vi "Trajectory Builder.vi"() -> ()   [LabVIEW 2023]
uses:
  Types/Limits.ctl
  Types/Overrides.ctl
  Types/Trajectory Data.ctl
  Types/Segment Type.ctl
  Types/Path Type.ctl
  Types/Drive Type.ctl
  Types/Angluar Limits.ctl
  Types/Command Editor Info.ctl
  Types/Single Cmd Info.ctl
  <vilib>/picture/picture.llb/imagedata.ctl
  <vilib>/Utility/miscctls.llb/LVPositionTypeDef.ctl
  <vilib>/Utility/miscctls.llb/LVRowAndColumnTypeDef.ctl
  Types/Internal Path Stuff.ctl
  <vilib>/Utility/miscctls.llb/LVBoundsTypeDef.ctl
  <vilib>/event_ctls.llb/lveventtype.ctl
  Global Settings.vi
panel:
  in  "Push":bool
  out "Picture":picture
  out "C":bool
  in  "Cache":T4
  out "Trajectory Data":T5
  out "CU":bool
  in  "Zero Velocity":bool
  in  "Reverse Path":bool
  in  "Robot Backwards":bool
  out "Duration (s)":dbl format="%#.4g"
  out "Distance (ft)":dbl format="%#.1g"
  in  "Instructions":string="Directions:\nUse mouse to ...\n    move robot position (rectangle with arrow)\n    rotate robot (red arrow)\n    move waypoints (numbered circles)\nClick in open space to add a waypoint\nShift click to delete a waypoint\nHover over a waypoint and use arrow keys to nudge\n\nTime slider and Play button will run robot along path to test for collisions.\n\nNew creates a new path at default location\n\nAppend creates a path using current path's position and heading.\n\nTo add a command, move robot using Time slider and double click the Command in Palette.\n\nYou can modify command timing in the graph or Command Sequencer tree.\n\nEnable/disable a command by clicking on the enable column item.\n\nDelete a command by shift-clicking in the enable column.\n\nTo configure command parameters, Select the command name in the tree, Open Panel, enter parameters, and Inhale the parameters.\n\nYou may sometimes want to type values into WayPoints directly.\n\nOverrides allow you to set accel and V limits for any turn."
  out "Command Palette":picture
  in  "Directory":bool
  in  "Tab Control":T7(tab)
  in  "Angular Limits":T8={"Velocity (deg/s)"=6.0, "Accel (deg/s^2)"=360.0, "Jerk (deg/s^3)"=1000.0} {"Jerk (deg/s^3)" min=0.01 step=1.0; "Accel (deg/s^2)" min=0.01; "Velocity (deg/s)" min=0.01}
  in  "Path Type":T9=enum."Bezier"
  in  "Overrides":T10=[{"Count"="1", "Angular Override"=0.0, "Enabled?"=FALSE, "Velocity Override"=6.0, "Angle Override"=nan}] {"Angle Override" step=5.0; "Velocity Override" step=5.0; "Angular Override" step=5.0}
  in  "Center Flip":bool
  in  "Sample Period (s)":dbl=0.02 min=0.001 max=1.0 format="%#_6p"
  in  "Limits":T11={"Velocity (fps)"=6.0, "Accel (fps^2)"=15.0, "Jerk (fps^3)"=150.0, "StoopidFast (fps)"=6.0} {"StoopidFast (fps)" min=0.01; "Jerk (fps^3)" min=0.01 step=1.0; "Accel (fps^2)" min=0.01; "Velocity (fps)" min=0.01}
  in  "Conditions":T12 {"vFinal (fps)" min=0.0; "vInitial (fps)" min=0.0}
  in  "Drive Type":T13=enum."Holonomic"
  in  "WayPoints":cluster{"x":dbl, "y":dbl, "th":dbl}[](array[cluster])
  in  "Turn Angle Limit (deg)":dbl=90.0
  in  "Allow Angles > 90":bool=TRUE
  in  "Stoopid Overlap %":dbl min=0.0
  in  "Unjank":bool
  in  "Turn Deceleration":bool=TRUE
  in  "Turn Acceleration":bool=TRUE
  in  "Open Command":bool
  in  "Inhale":bool
  in  "Command Sequence":string(tree)
  in  "Projects":u16(ring) items=["2024 Crescendo Robot Project.lvproj"]
  in  "Refresh":bool
  in  "Snap to foot":bool
  in  "Angle Limiter":enum16{"90", "45", "15", "1"}(ring)=enum."15"
  in  "Snap robot to baseline":bool
  in  "Background":u16(ring) items=["C Field", "CU Field", "RR Field", "IR Field", "Barrels", "Bounce", "Slalom", "Galactic Search A", "Galactic Search B"]
  in  "Robot Color":u32(colorbox)=14421504
  out "Field Size (ft)":cluster{"width":dbl, "height":dbl}={"width"=26.9167, "height"=35.2142} {"width" format="%#.1g"; "height" format="%#.1g"}
  in  "Robot Size (in)":cluster{"width":dbl, "height":dbl}={"width"=28.0, "height"=28.0}
  in  "Hide Path":bool
  in  "Time (s)":dbl(slide) scale=0.0..3.1199999999999997 scale format="%#.1g"
  in  "Play":bool
  out "fps":dbl[](graph)
  in  "Append":bool
  in  "Open":i32(listbox)
  in  "Filename":string
  in  "Save":bool
  in  "New":bool
  out "slalom":bool
  out "barrels":bool
  out "bounce":bool
  out "G-S B":bool
  out "G-S A":bool
  out "RR":bool
  out "IRR":bool
  # "Command Palette"
  # "StupidFast makes each linear segment into a\nvelocity ramp to max speed (for clothoid paths only)"
  # "Nicotine"
  # "A"
  # "V"
  # "O"
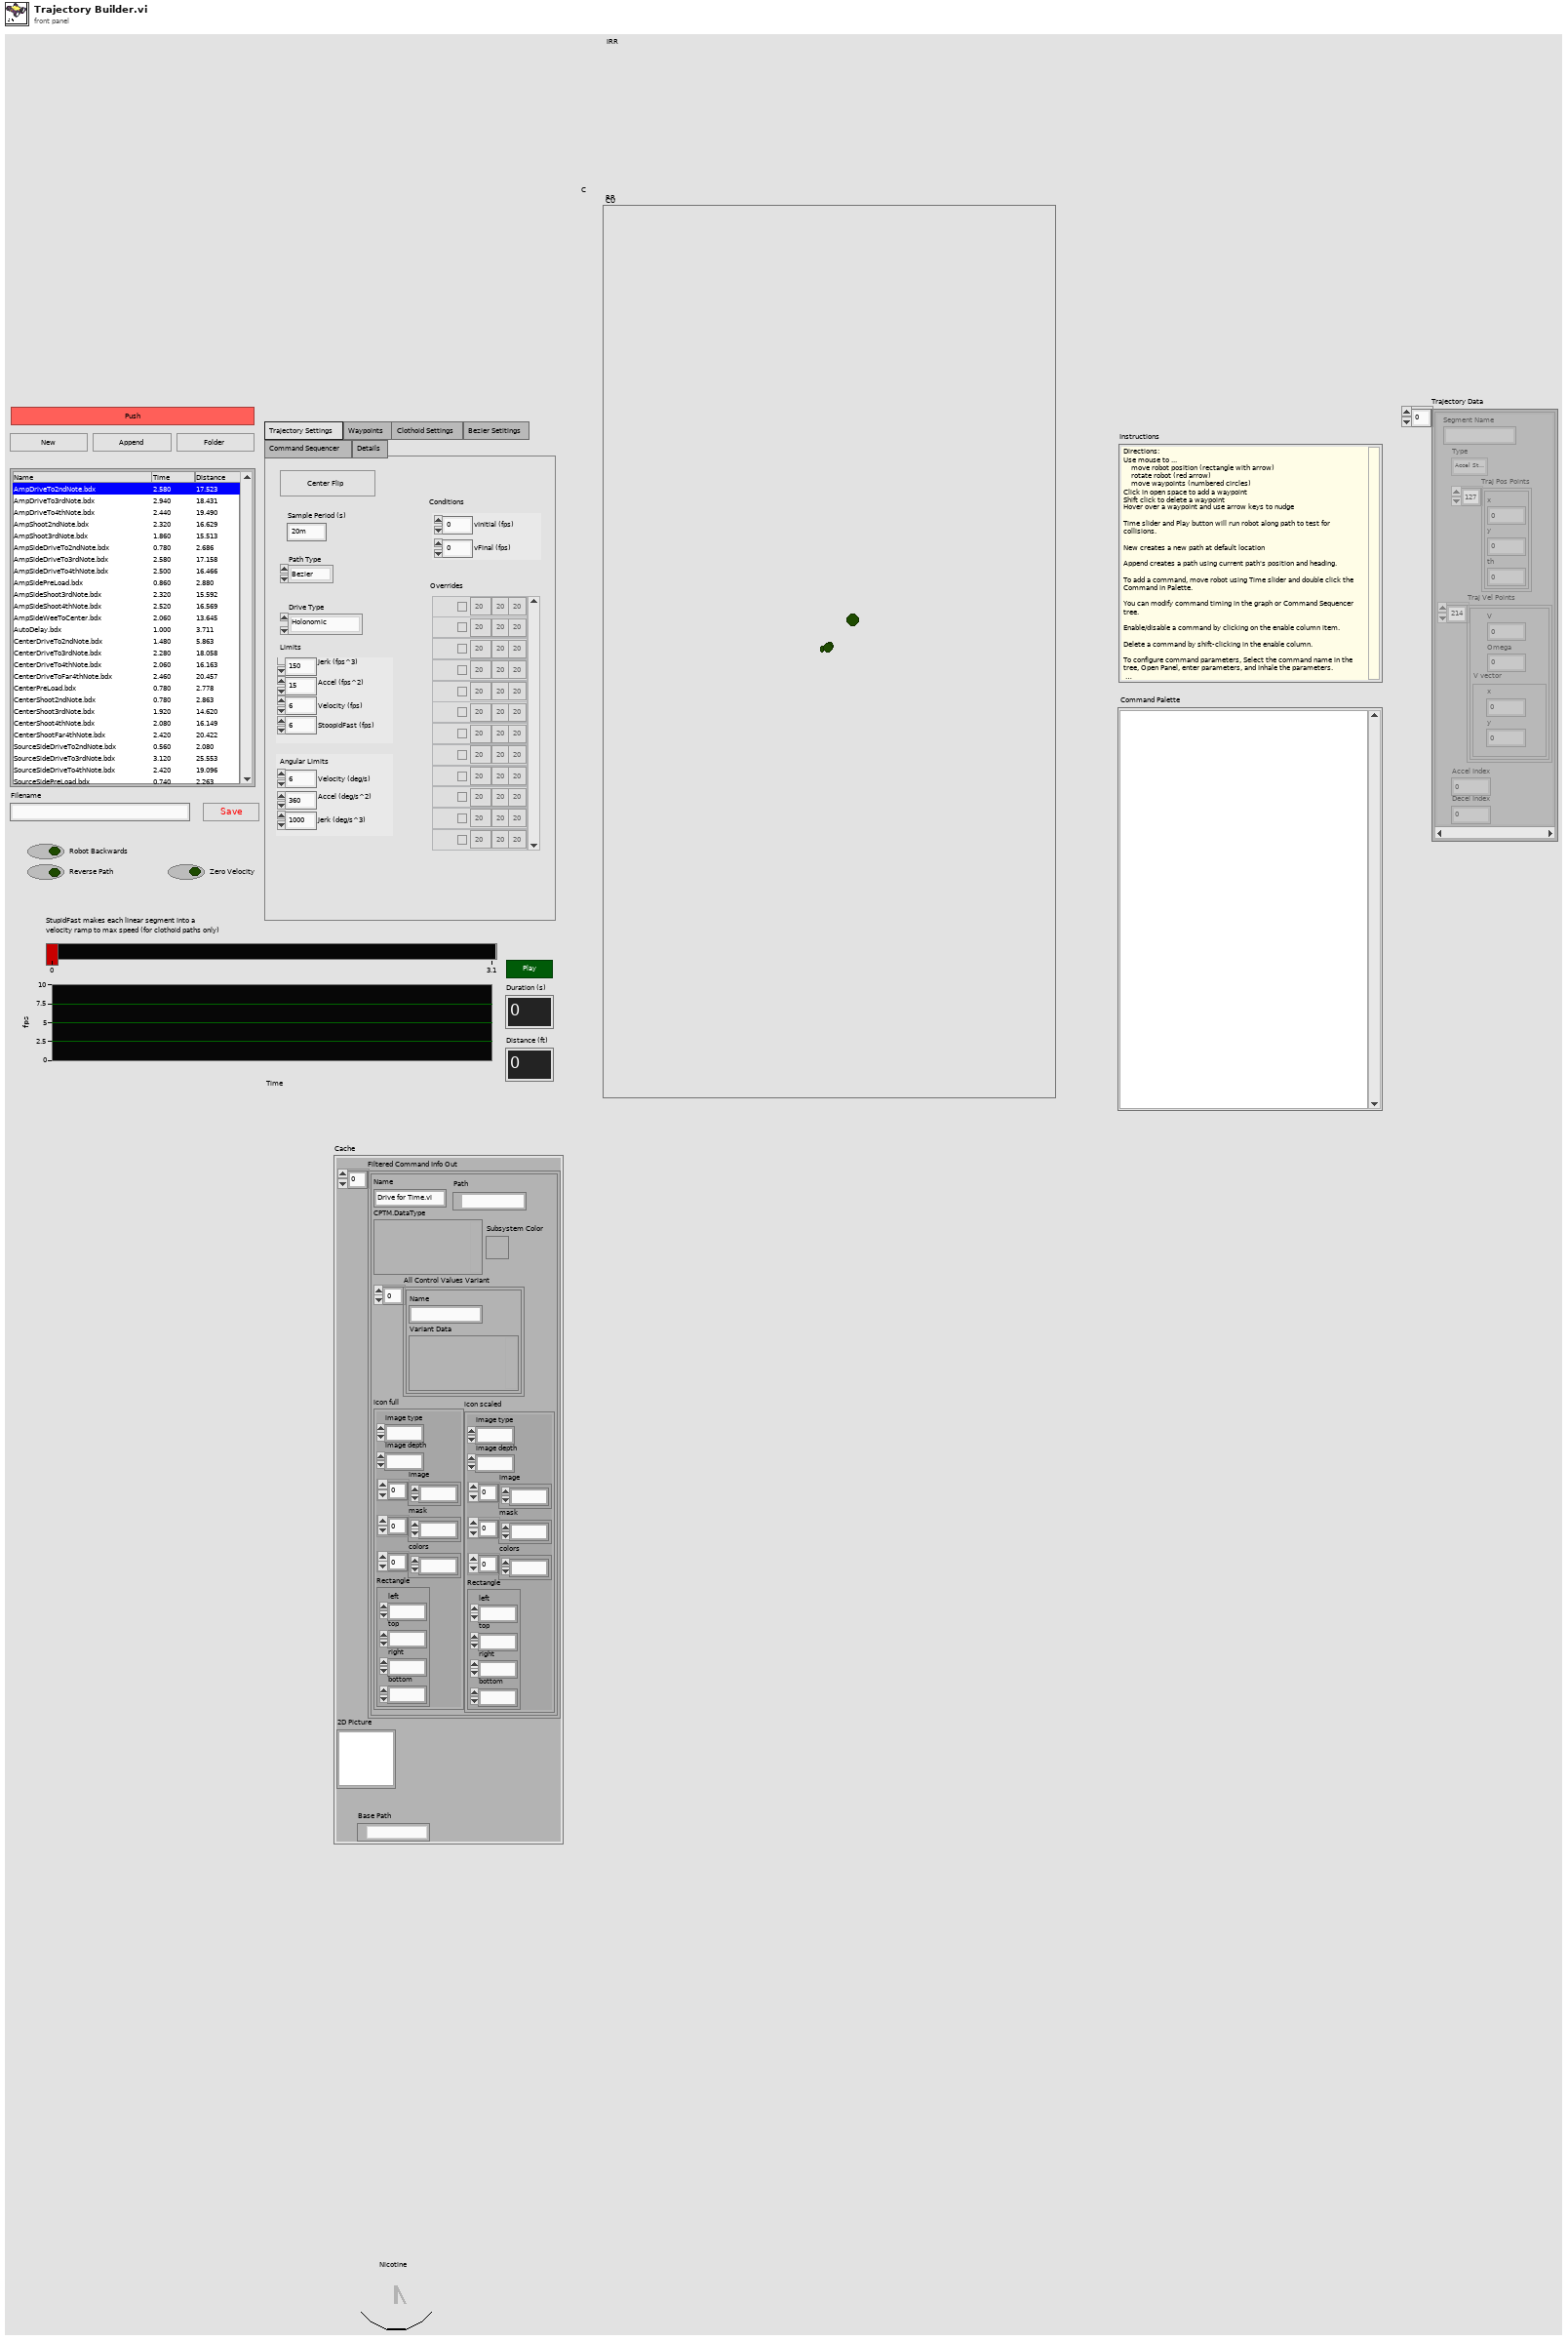
[diagram p1: front panel]
types:
  T1 = typedef "Command Editor Info.ctl" = T2[]
  T2 = typedef "Single Cmd Info.ctl" = cluster{"Name":string, "CPTM.DataType":variant, "All Control Values Variant":cluster{"Name":string, "Variant Data":variant}[], "icon full":T3, "icon scaled":T3, "Path":path, "Subsystem Color":u32}
  T3 = typedef "imagedata.ctl" = cluster{"image type":i32, "image depth":i32, "image":u8[], "mask":u8[], "colors":u32[], "Rectangle":cluster{"left":i16, "top":i16, "right":i16, "bottom":i16}}
  T4 = cluster{"Filtered Command Info Out":T1, "2D Picture":picture, "Base Path":path}
  T5 = typedef "Trajectory Data.ctl" = cluster{"Segment Name":string, "Type":T6, "Traj Pos Points":cluster{"x":dbl, "y":dbl, "th":dbl}[], "Traj Vel Points":cluster{"V":dbl, "Omega":dbl, "V vector":cluster{"y":dbl, "x":dbl}}[], "Accel Index":i32, "Decel Index":i32}[]
  T6 = typedef "Segment Type.ctl" = enum16{"Accel Straight", "Const Straight", "Blend", "Circle", "Bezier"}
  T7 = enum32{"Trajectory Settings", "Waypoints", "Clothoid Settings", "Bezier Setitings", "Command Sequencer", "Details"}
  T8 = typedef "Angluar Limits.ctl" = cluster{"Velocity (deg/s)":dbl, "Accel (deg/s^2)":dbl, "Jerk (deg/s^3)":dbl}
  T9 = typedef "Path Type.ctl" = enum16{"Clothoid", "Bezier"}
  T10 = typedef "Overrides.ctl" = cluster{"Count":string, "Angular Override":dbl, "Enabled?":bool, "Velocity Override":dbl, "Angle Override":dbl}[]
  T11 = typedef "Limits.ctl" = cluster{"Velocity (fps)":dbl, "Accel (fps^2)":dbl, "Jerk (fps^3)":dbl, "StoopidFast (fps)":dbl}
  T12 = cluster{"vInitial (fps)":dbl, "vFinal (fps)":dbl}
  T13 = typedef "Drive Type.ctl" = enum16{"Nonholonomic", "Holonomic"}
  T14 = cluster{"Sample Period (s)":dbl, "Limits":T11, "Conditions":cluster{"vInitial (fps)":dbl, "vFinal (fps)":dbl}, "Overrides":T10, "Angular Limits":T8}
  T15 = typedef "LVRowAndColumnTypeDef.ctl" = cluster{"Row":i32, "Column":i32}
  T16 = typedef "LVPositionTypeDef.ctl" = cluster{"Left":i32, "Top":i32}
  T17 = cluster{"Index":i32, "Pt Test Results":enum16{"Miss", "Rect Hit", "Arrow Hit"}}
  T18 = cluster{"Drag Object":cluster{"Index":i32, "x":dbl, "y":dbl}, "Hover Object":cluster{"Index":i32, "Pt Test Results":enum16{"Miss", "Rect Hit", "Arrow Hit"}}, "Filename":string}
  T19 = cluster{"Trajectory Data":T5, "Points":cluster{"x":dbl, "y":dbl, "th":dbl}[], "output cluster":cluster{"Sample Period (s)":dbl, "Limits":T11, "Conditions":cluster{"vInitial (fps)":dbl, "vFinal (fps)":dbl}, "Overrides":T10, "Angular Limits":T8}, cluster{"Time (s)":dbl, T2, bool}[]}
  T20 = typedef "Internal Path Stuff.ctl" = cluster{"Trajectory Data":T5, "Updated Waypoints":cluster{"x":dbl, "y":dbl, "th":dbl}[], cluster{"Sample Period (s)":dbl, "Limits":T11, "Conditions":cluster{"vInitial (fps)":dbl, "vFinal (fps)":dbl}, "Overrides":T10, "Angular Limits":T8}, "Commands out":cluster{"Time (s)":dbl, T2, bool}[]}
  T21 = typedef "LVBoundsTypeDef.ctl" = cluster{"Width":u32, "Height":u32}
  T22 = typedef "lveventtype.ctl" = enum32{"Null", "Timeout", "Annotation Menu Selection", "Annotation Menu Selection?", "App Instance Close", "App Instance Close?", "Autoscale Range Change", "Bookmark Info Change", "Cell Edit", "Cell Edit?", "Cursor Grab", "Cursor Grab?", "Cursor Menu Selection", "Cursor Menu Selection?", "Cursor Move", "Cursor Release", "Data Change", "Direction Change", "Display State Change", "Drag Ended", "Drag Enter", "Drag Leave", "Drag Over", "Drag Source Update", "Drag Starting", "Drag Starting?", "Drop", "Exec State Change", "Key Down", "Key Down?", "Key Repeat", "Key Repeat?", "Key Up", "Listbox Double Click", "Menu Activation?", "Menu Selection (App)", "Menu Selection? (App)", "Menu Selection (User)", "Mouse Down", "Mouse Down?", "Mouse Enter", "Mouse Leave", "Mouse Move", "Mouse Up", "Mouse Wheel", "NI Security User Change (App)", "Pane Size", "Panel Close", "Panel Close?", "Panel Resize", "Plot Attribute Change", "Scale Range Change", "Shortcut Menu Activation?", "Shortcut Menu Selection (App)", "Shortcut Menu Selection? (App)", "Shortcut Menu Selection (User)", "Tree Double Click", "Tree Drag", "Tree Drag?", "Tree Drop", "Tree Drop?", "Tree Item Close", "Tree Item Close?", "Tree Item Open", "Tree Item Open?", "User Event", "Value Change"}
  T23 = enum32{"Invalid", "Standard", "Closed", "Hidden", "Minimized", "Maximized"}
  T24 = cluster{"width":dbl, "height":dbl, "width":dbl, "height":dbl}
  T25 = cluster{"Robot Backwards":bool, "Reverse Path":bool}
  T26 = cluster{cluster{"Robot Backwards":bool, "Reverse Path":bool}, "Trajectory Data":T5, "Commands out":cluster{"Time (s)":dbl, T2, bool}[], cluster{"Sample Period (s)":dbl, "Limits":T11, "Conditions":cluster{"vInitial (fps)":dbl, "vFinal (fps)":dbl}, "Overrides":T10, "Angular Limits":T8}, "Updated Waypoints":cluster{"x":dbl, "y":dbl, "th":dbl}[], "Time & Dist":cluster{"Time (s)":dbl, "Distance (ft)":dbl}, "Zero Velocity":bool, cluster{"Drive Type":T13, "Path Type":T9}}
  T27 = cluster{"Trajectory Data":T5, "Updated Waypoints":cluster{"x":dbl, "y":dbl, "th":dbl}[], cluster{"Sample Period (s)":dbl, "Limits":T11, "Conditions":cluster{"vInitial (fps)":dbl, "vFinal (fps)":dbl}, "Overrides":T10, "Angular Limits":T8}, "Commands out":cluster{"Time (s)":dbl, T2, bool}[]}
  T28 = cluster{"Sample Period (s)":dbl, cluster{"Velocity (fps)":dbl, "Accel (fps^2)":dbl, "Jerk (fps^3)":dbl, "StoopidFast (fps)":dbl}, "Conditions":cluster{"vInitial (fps)":dbl, "vFinal (fps)":dbl}, "Overrides":T10, "Angular Limits":T8}
  T29 = cluster{"Velocity (fps)":dbl, "Accel (fps^2)":dbl, "Jerk (fps^3)":dbl, "StoopidFast (fps)":dbl}
  T30 = cluster{"Trajectory Data":T5, "Points out":cluster{"x":dbl, "y":dbl, "th":dbl}[], "Fields":cluster{"Sample Period (s)":dbl, cluster{"Velocity (fps)":dbl, "Accel (fps^2)":dbl, "Jerk (fps^3)":dbl, "StoopidFast (fps)":dbl}, "Conditions":cluster{"vInitial (fps)":dbl, "vFinal (fps)":dbl}, "Overrides":T10, "Angular Limits":T8}, "Commands out":cluster{"Time (s)":dbl, T2, bool}[]}
  T31 = typedef "LVPoint32TypeDef.ctl" = cluster{"Horizontal":i32, "Vertical":i32}
  T32 = cluster{"Shift":bool, "Ctrl":bool, "Alt":bool, "Cmd":bool, "Opt":bool}
  T33 = cluster{"Snap robot to baseline":bool, "Snap to foot":bool, "Angle Limiter":enum16{"90", "45", "15", "1"}}
  T34 = cluster{i32, "Pt Test Results":enum16{"Miss", "Rect Hit", "Arrow Hit"}}
  T35 = typedef "eventvkey.ctl" = enum16{"ASCII", "Enter", "Return", "Shift", "Ctrl", "Alt", "Cmd", "Opt", "Caps", "NumLock", "Clear", "Break", "Up", "Down", "Left", "Right", "Insert", "Delete", "Home", "End", "PageUp", "PageDown", "Escape", "Help", "Pause", "ScrollLock", "F1", "F2", "F3", "F4", "F5", "F6", "F7", "F8", "F9", "F10", "F11", "F12", "F13", "F14", "F15", "F16", "F17", "F18", "F19", "F20", "F21", "F22", "F23", "F24", "Play", "VolumeUp", "VolumeDown", "Mute", "Two Byte Char"}
  T36 = cluster{"Name":string, "CPTM.DataType":variant, "Get All Control Values Variant":cluster{"Name":string, "Variant Data":variant}[], "Color 256":T3, "Subsystem Color":u32}[]
  T37 = cluster{"Filtered Command Info Out":T1, "2D Picture":picture, "stripped path":path}
  T38 = cluster{"Horizontal":dbl, "Vertical":dbl, "th":dbl}
  T39 = cluster{"Name":string, "Color":u32, "Style":i32, "Point Style":i32, "Name Visible":bool, "Allow Drag":bool, "Annotation Mode":i32, "Plot":i32, "Index":i32, "Position":cluster{"X":dbl, "Y":dbl}, "X Scale":i32, "Y Scale":u32, "Show Arrow":bool, "Lock Name":bool, "Plot Area":i32, "Label Offset":cluster{"X":dbl, "Y":dbl}}[]
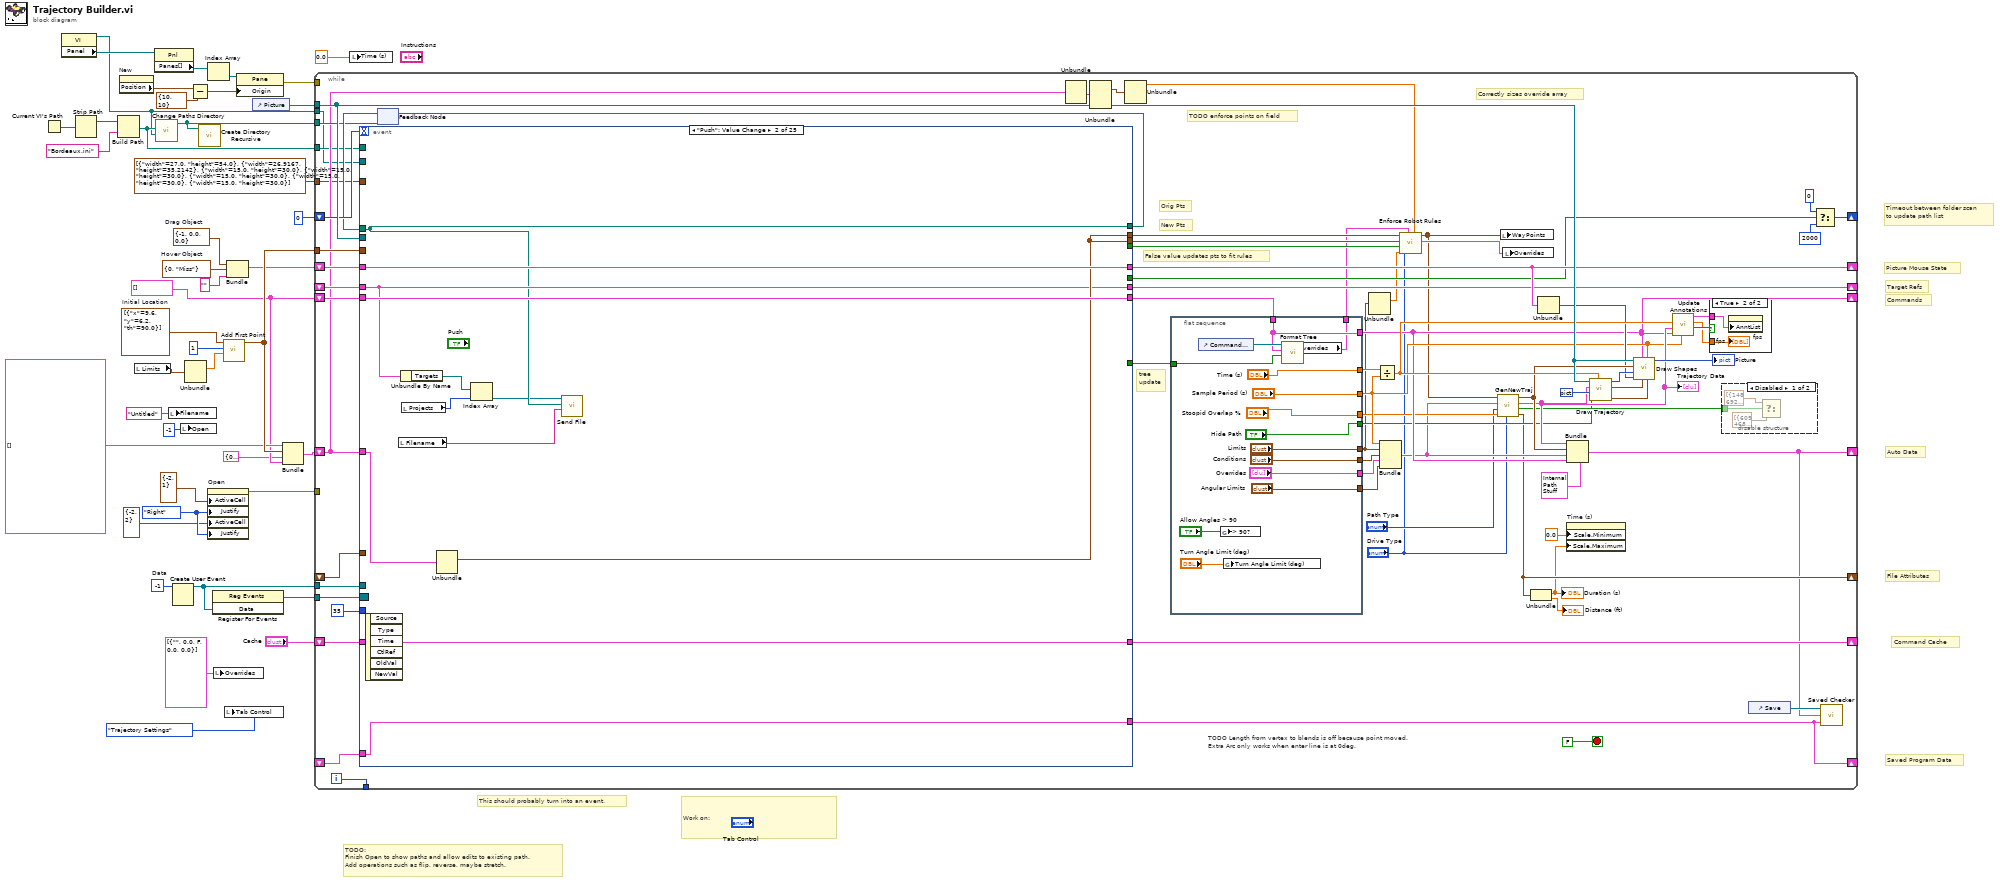
[diagram p0: block diagram]
diagram:
  w10 = enum16{"Left", "Center", "Right"}."Right" ("Active Cell:Cell Justification")
  w17 = cluster{"Time (s)":dbl, T2, bool}[] []
  w31 = -1  # Data
  w28 = T17 {"Index"=0, "Pt Test Results"=enum."Miss"}  # Hover Object
  w27 = cluster{"Index":i32, "x":dbl, "y":dbl} {"Index"=-1, "x"=0.0, "y"=0.0}  # Drag Object
  w40 = cluster{"x":dbl, "y":dbl, "th":dbl}[] [{"x"=9.6, "y"=6.2, "th"=90.0}]  # Initial Location
  # "Saved Program Data"
  # "Command Cache"
  # "File Attributes"
  # "Commands"
  # "Target Refs"
  # "Picture Mouse State"
  # "Auto Data"
  # "Timeout between folder scan\nto update path list"
  # "This should probably turn into an event."
  # "Work on:"
  # "TODO: \nFinish Open to show paths and allow edits to existing path.\nAdd operations such as flip, reverse, maybe stretch."
  n1 = Current VI's Path() -> (path=w15:path)
  n2 = property class="VI"() -> (reference out=w6:refnum<vi>, "Panel"=w25:refnum<vi>)  [unwired: 2 in, 1 out]
  n3 = Strip Path(path=w15) -> (stripped path=w14:path)  [unwired: 1 out]
  n4 = Build Path(base path=w14, name or relative path="Bordeaux.ini" ("format string")) -> (appended path=w8:path)
  n5 = property on="New" class="Bool"() -> ("Position"=w21:T16)  [unwired: 2 in, 2 out]
  n6 = local read "Limits"() -> (w37:T11)
  n7 = property class="Pnl"(reference=w25) -> ("Panes[]"=w24:refnum<vi>[])  [unwired: 1 in, 2 out]
  n8 = call "Change Paths Directory.vi"("VI Refnum"=w6, "config path"=w8) -> ("Bordeaux paths out"=w7:path)  [unwired: 9 in]
  n9 = local write "Filename"("Untitled" ("Filename")) -> ()
  n10 = Create User Event(user event datatype=w31) -> (user event=w32:refnum<user-event>)  [unwired: 1 in, 1 out]
  n11 = local write "Open"(-1) -> ()
  n12 = Unbundle(w37) -> ("Accel (fps^2)"=w36:dbl)  [unwired: 3 out]
  n13 = Subtract(x=w21, y=T16 {"Left"=10, "Top"=10}) -> (x-y=w20:T16)
  n14 = call <vilib>:"Create Directory Recursive.vi"("directory"=w7) -> ()  [unwired: 4 in, 3 out]
  n15 = Index Array(array=w24) -> (element=w23:refnum<vi>)  [unwired: 1 in]
  n16 = property on="Open" class="MCListbox (strict)"("ActiveCell"=T15 {"Row"=-2, "Column"=1} ("Active Cell:Active Cell"), "Justify"=w10, "ActiveCell"=T15 {"Row"=-2, "Column"=2} ("Active Cell:Active Cell"), "Justify"=w10) -> (error out=w11:errorcluster)  [unwired: 2 in, 1 out]
  n17 = register-events(w32) -> (reference out=w33:refnum<event-registration>)  [unwired: 2 in, 1 out]
  n18 = local write "Overrides"(T10 [{"Count"="", "Angular Override"=0.0, "Enabled?"=FALSE, "Velocity Override"=0.0, "Angle Override"=0.0}] ("Overrides")) -> ()
  n19 = call "Add First Point.vi"("Accel (f/s^2)"=w36, "Time (s)"=1 ("th"), "Initial Points"=w40) -> ("Points"=w30:cluster{"x":dbl, "y":dbl, "th":dbl}[])  [unwired: 8 in]
  n20 = local write "Tab Control"(T7."Trajectory Settings" ("Tab Control")) -> ()
  n21 = Bundle("Drag Object"=w27, "Hover Object"=w28, "Filename"="") -> (w26:T18)  [unwired: 1 in]
  n22 = property class="Pane"(reference=w23, "Origin"=w20) -> (error out=w19:errorcluster)  [unwired: 1 in, 1 out]
  n23 = control-ref of="Picture"() -> (w42:refnum<vi>)
  n24 = Bundle("Trajectory Data"=T5 [], "Points"=w30, "output cluster"=T14 {"Sample Period (s)"=0.2, "Limits"={"Velocity (fps)"=6.0, "Accel (fps^2)"=32.0, "Jerk (fps^3)"=1500.0, "StoopidFast (fps)"=12.0}, "Conditions"={"vInitial (fps)"=0.0, "vFinal (fps)"=0.0}, "Overrides"=[], "Angular Limits"={"Velocity (deg/s)"=0.0, "Accel (deg/s^2)"=0.0, "Jerk (deg/s^3)"=0.0}}, w17) -> (w4:T19)  [unwired: 1 in]
  n25 = while {
    tunnel: w30 -> [w114]
    tunnel: w42 -> [w113]
    shift-right: [w86] -> _
    shift-left: 0 -> [w107]
    shift-right: [w55] -> _
    shift-left: _ -> [w106]
    tunnel: w7 -> [w93]
    tunnel: w33 -> [w101]
    tunnel: w32 -> [w100]
    shift-right: [w98] -> _
    shift-left: _ -> [w99]
    shift-right: [w50] -> _
    shift-left: w4 -> [w70]
    shift-right: [w90] -> _
    shift-left: w26 -> [w91]
    shift-right: [w82] -> _
    shift-left: _ -> [w81]
    shift-right: [w79] -> _
    shift-left: "Cache" -> [w80]
    shift-right: [w72] -> _
    shift-left: w17 -> [w77]
    tunnel: w19 -> [_]
    tunnel: cluster{"width":dbl, "height":dbl}[] [{"width"=27.0, "height"=54.0}, {"width"=26.9167, "height"=35.2142}, {"width"=15.0, "height"=30.0}, {"width"=15.0, "height"=30.0}, {"width"=15.0, "height"=30.0}, {"width"=15.0, "height"=30.0}, {"width"=15.0, "height"=30.0}] -> [w67]
    tunnel: [w64] -> _
    tunnel: w11 -> [_]
    tunnel: w8 -> [w58]
    tunnel: w6 -> [w57]
    i -> [w64]
    stop <- FALSE stop-if-true
    # "False value updates pts to fit rules"
    # "tree\nupdate"
    # "New Pts"
    # "Orig Pts"
    # "Correctly sizes override array"
    # "TODO Length from vertex to blends is off because point moved.\nExtra Arc only works when enter line is at 0deg."
    # "TODO enforce points on field"
    n26 = feedback #1(w93) -> (w94:path)
    n27 = event shown="[1] \"Push\": Value Change" {
      selector: w101 -> [_ _ _ _ _ _ _ _ _ _ _ _ _ _ _ _ _ _ _ _ _ _ _ _ _]
      dyn-events: _ -> [_ _ _ _ _ _ _ _ _ _ _ _ _ _ _ _ _ _ _ _ _ _ _ _ _]
      timeout: w107 -> [_ _ _ _ _ _ _ _ _ _ _ _ _ _ _ _ _ _ _ _ _ _ _ _ _]
      tunnel: [w167 w188 w203 w221 w227 w242 w265 w280 w288 w323 w430 w475 w516 w541 w566 w591 w595 w614 w655 w704 w738 w787 w813 w845 w876] -> w105
      tunnel: w114 -> [_ _ w203 _ _ _ _ _ _ _ _ _ _ _ _ _ _ _ _ _ _ _ _ _ _]
      tunnel: w113 -> [_ _ _ _ _ _ _ _ _ w322 w416 _ w503 _ _ _ _ _ _ _ _ _ _ _ _]
      tunnel: w94 -> [w165 w184 w201 w210 w232 w239 w257 w276 w287 w320 w427 w470 w517 w556 w569 w593 w601 w618 w659 w710 w743 w791 w818 w850 w881]
      tunnel: [w167 w188 w198 w221 w227 w242 w265 w280 w288 w317 w424 w467 w501 w541 w566 w591 w595 w614 w655 w704 w738 w787 w813 w845 w876] -> w104
      tunnel: w106 -> [_ _ _ _ _ w237 _ _ _ _ _ _ _ _ _ _ _ _ _ _ _ _ _ _ _]
      tunnel: [_ _ _ _ _ _ _ _ _ _ _ TRUE ("Flip Over Center") _ _ _ _ _ _ _ _ _ _ _ _ _] -> w56
      tunnel: [w165 w184 w201 w210 w232 w239 w257 w269 w287 w320 w427 w470 w517 w556 w569 w593 w601 w618 w659 w710 w743 w791 w818 w850 w881] -> w95
      tunnel: w100 -> [_ _ _ _ w231 _ _ _ _ _ _ _ _ w536 _ _ _ _ _ _ _ _ _ _ _]
      tunnel: [w169 w193 w200 w211 w230 w253 w267 w282 w295 w319 w426 w469 w504 w553 w568 w594 w600 w617 w658 w709 w742 w790 w817 w849 w880] -> w98
      tunnel: w99 -> [w169 w193 w200 w211 w230 _ w267 w282 _ w319 w426 w469 w504 w553 w568 w594 w600 w617 w658 w709 w742 w790 w817 w849 w880]
      tunnel: w70 -> [w168 w189 w199 w209 w228 w252 w266 w281 _ w318 w425 w468 w502 w542 w567 w592 _ w615 w656 w706 w739 w788 w814 w846 w877]
      tunnel: w91 -> [w166 w192 w197 w207 w226 w251 w262 w283 w303 w314 w417 w466 w499 w540 w565 w590 w599 w613 w654 w708 w741 w773 w816 w848 w879]
      tunnel: [w166 w192 w197 w207 w226 w251 w263 w283 w303 w316 w421 w466 w499 w540 w565 w590 w599 w613 w654 w708 w741 w774 w816 w848 w879] -> w90
      tunnel: [_ _ _ _ _ TRUE _ TRUE _ _ _ _ _ _ _ _ _ _ _ _ _ _ _ _ _] -> w85
      tunnel: [w164 w187 w195 w206 w225 w249 w256 w274 w302 w310 w419 w465 w497 w539 w560 w580 w598 w616 w657 w707 w740 w789 w815 w847 w878] -> w82
      tunnel: w81 -> [w164 w187 w195 w206 w225 w249 w256 w274 w302 w310 w419 w465 w497 w539 w563 w580 w598 w616 w657 w707 w740 w789 w815 w847 w878]
      tunnel: w80 -> [w163 w191 w196 w205 w224 w248 w255 w273 w301 w312 w418 w464 w496 w538 w562 _ w597 w602 w647 w697 w723 w771 w798 w836 w863]
      tunnel: [w163 w191 w196 w205 w224 w248 w255 w273 w301 w312 w418 w464 w496 w538 w562 w585 w597 w602 w647 w697 w723 w771 w798 w836 w863] -> w79
      tunnel: 35 -> [_ _ _ _ _ _ _ _ _ _ _ _ _ _ _ _ _ _ _ _ _ _ _ w838 w872]
      tunnel: w77 -> [w162 w190 _ w204 w223 w244 w264 w271 _ w311 w415 w463 w495 w537 w561 w584 w596 w603 w645 w702 w726 w776 w801 w837 w865]
      tunnel: [w162 w190 _ w204 w223 w244 w264 w271 w299 w311 w415 w463 w495 w537 w561 w584 w596 w603 w649 w703 w724 w776 w802 w837 w866] -> w76
      tunnel: [w161 _ TRUE _ _ _ _ _ TRUE _ _ _ _ _ _ _ _ w606 w648 TRUE w725 _ w800 _ TRUE] -> w75
      tunnel: w67 -> [w144 _ _ _ _ _ _ _ _ _ _ _ _ _ _ _ _ _ _ _ _ _ _ _ _]
      tunnel: w58 -> [_ _ _ _ _ _ _ w270 _ _ _ _ _ _ _ _ _ _ _ _ _ _ _ _ _]
      tunnel: w57 -> [_ _ _ _ _ _ _ w268 _ _ _ _ _ _ _ _ _ _ _ _ _ _ _ _ _]
      event Timeout; "Background", "Robot Color", "Robot Size (in)": Value Change {
        # "Occasionally update the listbox with all files in\nthe folder.\nAlso update the size of the picture, which field button\nis shown, color of the robot arrow,"
        n28 = event-data() -> ()  [unwired: 1 in, 1 out]
        n29 = Unbundle(w168) -> ("Updated Waypoints"=w167:cluster{"x":dbl, "y":dbl, "th":dbl}[])  [unwired: 3 out]
        n30 = call <vilib>:"Recursive File List.vi"("pattern"="*.bdx", "Folder Path"=w165) -> ("error out"=w170:errorcluster, "All Files in Dir"=w172:path[])  [unwired: 5 in, 3 out]
        n31 = Divide(x="Robot Size (in)", y=24.0 ("width")) -> (x/y=w157:cluster{"width":dbl, "height":dbl})
        n32 = for {
          tunnel: w172 -> [w179] mode=indexing
          tunnel: [w181] -> w171 mode=indexing
          tunnel: w170 -> [_]
          w173 = "%.3f" ("format string")
          n33 = call "Versioned Load.vi"("path"=w179) -> ("Overall"=w178:cluster{"Time (s)":dbl, "Distance (ft)":dbl})  [unwired: 3 in, 7 out]
          n34 = Strip Path(path=w179) -> (name=w180:string)  [unwired: 1 out]
          n35 = Unbundle(w178) -> ("Time (s)"=w177:dbl, "Distance (ft)"=w176:dbl)
          n36 = Format Into String(format string=w173, w177) -> (resulting string=w175:string)  [unwired: 2 in, 1 out]
          n37 = Format Into String(format string=w173, w176) -> (resulting string=w174:string)  [unwired: 2 in, 1 out]
          n38 = Build Array(w180, w175, w174) -> (w181:string[])
        }
        n39 = Negate(x=w157) -> (-x=w158:cluster{"width":dbl, "height":dbl})
        n40 = Unbundle(w158) -> ("width"=w156:dbl, "height"=w155:dbl)
        n41 = Unbundle(w157) -> ("width"=w154:dbl, "height"=w153:dbl)
        n42 = Bundle("width"=w156, "height"=w155, "width"=w154, "height"=w153) -> (w152:T24)  [unwired: 1 in]
        n43 = global write "Global Settings.vi" "Robot Rect"(w152) -> ()
        n44 = Index Array(array=w144, index="Background") -> (element=w143:cluster{"width":dbl, "height":dbl})
        "Field Size (ft)" <- w143
        n45 = global write "Global Settings.vi" "Field Size"(w143) -> ()
        n46 = property on="Open" class="MCListbox (strict)"("ItemNames"=w171) -> ()  [unwired: 2 in, 2 out]
        n47 = Replace Array Subset(array=bool[] [FALSE, FALSE, FALSE, FALSE, FALSE, FALSE, FALSE, FALSE], new element=TRUE, index="Background") -> (w148:bool[])
        n48 = Index Array(array=w148) -> (element #1=→"C":bool, element #2=→"CU":bool, element #3=→"RR":bool, element #4=→"IRR":bool, element #5=→"barrels":bool, element #6=→"bounce":bool, element #7=→"slalom":bool, element #8=→"G-S A":bool, element #9=→"G-S B":bool)  [unwired: 9 in]
        n49 = Index Array(array=T21[] [{"Width"=614, "Height"=1215}, {"Width"=662, "Height"=864}, {"Width"=415, "Height"=835}, {"Width"=415, "Height"=835}, {"Width"=415, "Height"=835}, {"Width"=415, "Height"=835}, {"Width"=415, "Height"=835}], index="Background") -> (element=w146:T21)
        n50 = property on="Picture" class="Pict"("Draw Area Size"=w146) -> ()  [unwired: 2 in, 2 out]
        n51 = global write "Global Settings.vi" "Arrow Color"("Robot Color") -> ()
        n52 = First Call?() -> (First Call?: T/F=w161:bool)
      }
      event "Push": Value Change {
        n53 = event-data() -> ()  [unwired: 1 in, 6 out]
        n54 = local read "Filename"() -> (w182:string)
        n55 = Unbundle By Name(w187) -> ("Targets"=w186:refnum<vi>[])
        n56 = local read "Projects"() -> (w185:u16)
        n57 = Unbundle(w189) -> ("Updated Waypoints"=w188:cluster{"x":dbl, "y":dbl, "th":dbl}[])  [unwired: 3 out]
        n58 = Index Array(array=w186, index=w185) -> (element=w183:refnum<vi>)
        n59 = call "Send File.vi"("Filename"=w182, "Host Base Path"=w184, "TargetItem"=w183) -> ()  [unwired: 7 in, 2 out]